vi "HFRR ADV v039.vi"() -> ()   [LabVIEW 2025] (continued)
  # "Calibration completed successfully. The measured stroke length is within the acceptable tolerance range of the factory calibration value."
  # "Calibration failed. The measured stroke length differs from the factory calibration value by more than 20%. Please perform the calibration again."
  # "Step 1 — Ball Holder"
  # "Remove the ball holder by loosening and removing the center screw for Friction calibration."
  # "Step 2 — Disc Holder"
  # "Remove the disc holder by loosening and removing the opposing screws. Clean any fluid present in the disc holder."
  # "Step 3 — Calibration Head"
  # "Place the calibration holder in position and securely tighten the center screw."
  # "Step 4 — Calibration Holder"
  # "Place the calibration holder in position and tighten the two securing screws"
  # "Step 5 — Tare (Spring at Free Length)"
  # "Ensure the spring is at its contact (compressed) length — the micrometer head is in contact. Click Tare Sensor to zero the friction force baseline."
  # "Step 6 — Measure Friction Force"
  # "Run the Actual Test to measure Friction Force."
  # "Spring Constant: k = 1.000 N/mm\nSpring force |F| = k Ч d"
  # "Calibrates the sample/bath temperature sensor. \nUsed for test specimen and lubricant temperature measurement."
  # "Calibrates the ambient air temperature sensor. \nUsed for environmental chamber monitoring."
  # "Set B\n60 °C\nHigh-point calibration"
  # "Set A\n0 °C\nIce-point calibration"
  # "Set B\n60 °C\nHigh-point calibration"
  # "Set A\n0 °C\nIce-point calibration"
  # "Select Temperature Sensor"
  # "Choose which temperature sensor you are calibrating. Both use the same two-\npoint procedure: 0 °C (ice-point) and 60 °C (high-point)."
  # "Step 1 — Reference Instrument Setup"
  # "Connect a calibrated reference to the DUT port. This calibration performs two sets: one at 0 °C and one at 60 °C."
  # "Set A\n0 °C\nIce-point calibration"
  # "Set B\n60 °C\nHigh-point calibration"
  # "Allow the temperature bath to stabilise for at least 2 minutes at each set-point before recording the reading."
  # "Step 2 — Set A:  0 °C Calibration"
  # "Connect the  0 °C reference connector. Wait for the temperature to stabilise. Once stable, and click Record Point."
  # "Step 3 — Set B:  60 °C Calibration"
  # "Connect the  60 °C reference connector. Wait for the temperature to stabilise. Once stable, and click Record Point."
  # "Sample Temperature Calibration Complete"
  # "Sample Temperature Calibration PASSED\nMax deviation 0.200 °C — within ±0.5 °C tolerance. Two-point correction applied (0 °C & 60 °C)."
  # "Sample  Temperature Calibration Failed\nmeasured Sample Temperature differs from the factory calibration value"
  # "Step 1 — Reference Instrument Setup"
  # "Connect a calibrated reference to the DUT port. This calibration performs two sets: one at 0 °C and one at 60 °C."
  # "Set A\n0 °C\nIce-point calibration"
  # "Set B\n60 °C\nHigh-point calibration"
  # "Allow the temperature bath to stabilise for at least 2 minutes at each set-point before recording the reading."
  # "Step 2 — Set A:  0 °C Calibration"
  # "Connect the  0 °C reference connector. Wait for the temperature to stabilise. Once stable, and click Record Point."
  # "Step 3 — Set B:  60 °C Calibration"
  # "Connect the  60 °C reference connector. Wait for the temperature to stabilise. Once stable, and click Record Point."
  # "Air Temperature Calibration Complete"
  # "Sample Temperature Calibration PASSED\nMax deviation 0.200 °C — within ±0.5 °C tolerance. Two-point correction applied (0 °C & 60 °C)."
  # "Sample  Temperature Calibration Failed\nmeasured Sample Temperature differs from the factory calibration value"
  # "System Control Commands\nS;1 - Starts the full automation cycle (Runs Priming-humidify till 70RH sequence first, then switches to Maintenance).\nS;0 - Stops the system immediately and enters Standby mode (Safe State: All actuators OFF).\nM;1 - Skips the priming sequence and jumps directly to Maintenance mode (PID control).\nR;1 - Resets the logic state machine and clears all errors, returning to Standby.\nService Mode (Manual Control)\nX;1 - Enters Manual Service Mode. This disables all automatic logic, sensor safety checks, and timers.\nX;0 - Exits Manual Service Mode and returns to Standby (Safe State).\nActuator Commands (Only work after sending X;1)\nP;[0-255] - Sets the Pump PWM. Note that this is Active Low (0 = Max Flow, 255 = Pump OFF).\nF;I;[0-255] - Sets the Intake Fan speed (0 = OFF, 255 = Max Speed).\nF;O;[0-255] - Sets the Exhaust Fan speed (0 = OFF, 255 = Max Speed).\nD;1 - Turns the Dehumidifier Relay ON.\nD;0 - Turns the Dehumidifier Relay OFF."
  # "%RH"
  # "ISO : WS1.4"
  # "Start test and end test log--- done\nDisable heater ON and Humidity ON during the test --- done\ntemprature and ---done\nhumidity reach log\nauto start run true logic and log\nmanual start log once"
  # "Reference Fluid Information"
  # "Note:\nMake sure to place all images in the folder \"C:\\WinDucom\\im\" before clicking on \"Import Image.\""
  # "NOTE:\nPlace all the images in the path \"C:\\WinDucom\\im\" before clicking on Import Image"
  # "Wear Scar Measurements"
  # "Reference Fluid Information"
  # "Graph :"
types:
  T1 = enum32{"Home", "Dashboard", "Imaging", "Report", "Analysis", "About", "Test Setup", "Advance", "Calibration"}
  T2 = enum32{"HOME", "Test Setup", "Acquire", "Adv Scar", "Adv Scar Report", "Compare Files", "Calibration", "About", "Advance", "Mooha"}
  T3 = enum16{"ASTM D6079", "ISO 12156", "CEC F-096-A-06", "Custom"}
  T4 = enum32{"Dashboard 1", "Dashboard 2", "Dashboard 3"}
  T5 = enum32{"COF", "Friction", "ECR", "Temperature", "Stroke"}
  T6 = enum32{"Coefficient Of Friction", "Air Temperature", "Humidity", "Stroke", "Sample Temperature", "Electrical Contact Resistance", "Frequency", "Air Temp vs Rh"}
  T7 = enum32{"Main", "Stroke", "Friction", "Temperature"}
  T8 = enum32{"Stroke Calibration", "Friction Force Calibration", "Temperature Calibration", "Default"}
  T9 = enum32{"Step 1", "Step 2", "Step 3", "Step 4", "Step 5", "Step 6", "Step 7", "Step 8", "Step 9"}
  T10 = enum32{"Test Progress", "Stroke Points Completed"}
  T11 = enum32{"Page 1", "Page 2", "Page 3", "Page 4", "Page 5", "Page 6", "Page 7"}
  T12 = enum32{"Main", "Step 1", "Step 2", "Step 3", "Step 4", "Air Step 1", "Air Step 2", "Air Step 3", "Air Step 4"}
  T13 = enum32{"Air Temperature", "Sample Temperature", "Default"}
  T14 = enum32{"COMMUNICATION", "CALIBRATION", "Temp Variables", "Camera", "WO 2465 (1)", "WO 2465 (2)", "WO 2465 (3)"}
  T15 = typedef "Auto Start enum.ctl" = enum16{"Init", "Humidity & Temperature On", "Reach point", "Maintain Stage", "Start Stage", "close", "Exit"}
  T16 = typedef "imagedata.ctl" = cluster{"image type":i32, "image depth":i32, "image":u8[], "mask":u8[], "colors":u32[], "Rectangle":cluster{"left":i16, "top":i16, "right":i16, "bottom":i16}}
  T17 = enum32{"HOME", "Test Setup", "Acquire", "Compare Files", "Print Report", "About", "Advance", "Mooha"}
  T18 = cluster{"Read Heave and Surge":string, "Bytes at Heave Port":dbl, "Heave and Surge COM Port:":refnum<visa-resource-name>, "Com Port 2":refnum<visa-resource-name>, "Residual Due":string, "Heave COM Status 2":bool, "Heave COM Status":bool, "Port 2":bool, "Sway PPR":dbl, "Surge PPR":dbl, "Heave PPR":dbl, "Sway Pitch":dbl, "Surge Pitch":dbl, "Heave Pitch":dbl, "Sway Pulses/mm":dbl, "Surge Pulses/mm":dbl, "Heave Pulses/mm":dbl, "inner loop":dbl, "Read Heave and Surge 2":string, "String 36":string, "Write S":bool, "WriteCC1":string[], "Heave COM Loop":i32, "LastCom":string, "EXIT":bool, "Error Heave":errorcluster}
  T19 = enum8{"Enabled", "Disabled", "Disabled and Grayed Out"}
  T20 = cluster{"Read Uno":string, "Bytes at Heave Port":dbl, "UNO COM Port:":refnum<visa-resource-name>, "UNO COM Port: 2":refnum<visa-resource-name>, "Residual Due":string, "UNO COM Status 2":bool, "UNO COM Status":bool, "Port 2":bool, "Sway PPR":dbl, "Surge PPR":dbl, "Heave PPR":dbl, "Sway Pitch":dbl, "Surge Pitch":dbl, "Heave Pitch":dbl, "Sway Pulses/mm":dbl, "Surge Pulses/mm":dbl, "Heave Pulses/mm":dbl, "inner loop":dbl, "Read Heave and Surge 2":string, "String 36":string, "Write S":bool, "WriteCC1":string[], "Heave COM Loop":i32, "LastCom":string, "EXIT":bool, "Error Heave":errorcluster}
  T21 = enum32{"HOME", "Test Setup", "Acquire", "Adv Scar", "Adv Scar Report", "Compare Files", "About", "Advance", "Mooha"}
  T22 = typedef "POST ANALYSIS ENUM.ctl" = enum16{"OPEN EXE", "INIT", "OPEN FILE", "FIT", "DRAW REC", "DRAW LINE", "PAN", "ZOOM IN", "ZOOM OUT", "SET ZOOM", "CLEAR ROI", "GET MEASUREMENTS", "RESIZE MODE", "STREAM START", "STREAM STOP", "SHOW UI", "MINIMIZE UI", "HIDE UI", "CKISE APP", "CLOSE CONNECTION", "SAVE IMAGE", "SET ROI COLOR", "READ", "TCP CHECK", "CLOSE"}
  T23 = typedef "CAMERA LIVE FEED ENUM.ctl" = enum16{"OPEN EXE", "INIT", "READ", "CAMERA CONNECT", "CAMERA START", "CAMERA STOP", "CAMERA GRAY", "CAMERA RGB", "CAMERA MINIMIZE", "CAMERA CLOSE", "CAMERA MODE LIST", "CAMERA MODE SET", "CAMERA RESTORE", "CAMERA SAVE", "CLOSE"}
  T24 = enum16{"Always On", "Always Off", "Off While Running"}
  T25 = enum32{"Page 1", "Page 2", "Page 3", "Page 4", "Page 5", "Page 6"}
  T26 = enum32{"Home", "Dashboard", "Imaging", "Report", "Analysis", "About", "Test Setup", "Advance"}
  T27 = cluster{"File Name":string, "Test Method":string, "Operator":string, "Fuel Description":string, "Date and time":string}
  T28 = enum32{"Home", "Dashboard", "Imaging", "Report", "Analysis", "About", "Test Setup"}
  T29 = enum32{"HOME", "Test Setup", "Acquire", "Compare Files", "About", "Advance", "Mooha"}
  T30 = typedef "NI_ReportGenerationCore.lvlib/HTML Report Image Alignment.ctl" = enum16{"(default)", "LEFT", "RIGHT", "TOP", "TEXTTOP", "MIDDLE", "ABSMIDDLE", "BASELINE", "BOTTOM", "ABSBOTTOM"}
  T31 = cluster{"y":dbl, "LVDT STROKE DISPLAY":dbl, "y":dbl}
  T32 = enum16{"INIT", "READ", "MANUAL WRITE", "WRITE", "CLOSE", "ERROR INIT"}
diagram:
  w3 = 0.0 ("ch0_filt")
  w5 = -9999999.0 ("max_ch0")
  w6 = 9999999.0 ("min_ch0")
  w17 = FALSE ("Visible")
  w18 = T19."Enabled" ("Disabled")
  w21 = FALSE ("Visible")
  w20 = FALSE ("Humidity Off Command")
  w36 = "" ("USER ID")
  (unwired) T21."HOME" ("Main Tab")
  # "Temperature Continue Air Step 2"
  # "[CH1]    - FF\n[CH2]   - TEMPERATURE\n[CH3]    - Humidity\n[CH4]    - AIR TEMP\n[CH5]\\- Visa Uno\n[CH6] \\- Visa Due\n[CH7]  \\- file path\n[CH8]   - Displacement Gain\n[CHA]   - Stroke Gain\n[CHB]   - Stroke PID Gain\n[CHC]   -Language Selection\n[CHD]   -Power +\n[CHE]   -Power_\n[CHF]   -Heater\n[CHG]   -Humidity Wet\n[CHH]   -Humidity Dry\n[CHI]   -Integral Time \n[CHIJ   -Air intercept\n[CHI]   -Temp Intercept"
  n1 = local write "Cal Password"("" ("Cal Password")) -> ()
  n2 = property on="Auto Start Test" class="Bool (strict)"("Visible"=TRUE) -> ()  [unwired: 2 in, 2 out]
  n3 = property on="FRICVALZ 2" class="Bool (strict)"("DisabledEnum"=w18) -> ()  [unwired: 2 in, 2 out]
  n4 = property on="FRICVALZ 4" class="Bool (strict)"("DisabledEnum"=w18) -> ()  [unwired: 2 in, 2 out]
  n5 = property on="FRICVALZ 3" class="Bool (strict)"("DisabledEnum"=w18) -> ()  [unwired: 2 in, 2 out]
  n6 = property on="About" class="Clust (strict)"("Visible"=FALSE) -> ()  [unwired: 2 in, 2 out]
  n7 = property on="Wrong Password" class="Str"("Visible"=w17) -> ()  [unwired: 2 in, 2 out]
  n8 = property on="Calibration 2" class="TabCtl (strict)"("Visible"=w17) -> ()  [unwired: 2 in, 2 out]
  n9 = flat-sequence {
    tunnel: [w63] -> w2
    tunnel: [w108] -> w28
    tunnel: w2 -> [w103]
    tunnel: [w109] -> w30
    tunnel: w28 -> [w109]
    tunnel: w30 -> [w169]
    tunnel: [w169] -> w29
    tunnel: w29 -> [w200]
    tunnel: [w200] -> w39
    tunnel: w39 -> [w207]
    tunnel: [w213] -> w27
    tunnel: [w201] -> w26
    tunnel: [w255] -> w1
    tunnel: [w254] -> _
    tunnel: w27 -> [w254]
    tunnel: w26 -> [w255]
    frame #0 {
      n10 = call "CLOSE CONNECTION.vi"("error in (no error)"="error in (no error) 2") -> ("error out"=w68:errorcluster)  [unwired: 10 in]
      n11 = call <vilib>:"Clear Errors.vi"("error in (no error)"=w68) -> ("error out"=w67:errorcluster)  [unwired: 5 in, 1 out]
      n12 = disable-structure shown="Enabled" {
        disable-tunnel: w67 -> [w95 _]
        disable-tunnel: [w94 _] -> w66
        frame Enabled {
          n13 = call <userlib>:"Fit VI window to Largest Dec.vi"("error in (no error)"=w95, "border spacing (2 px)"=1) -> ("error out"=w98:errorcluster, "dup VI Ref"=w102:refnum<vi>)  [unwired: 4 in]
          n14 = invoke on="Invoke Node" class="VI" method="FP.Run-Time Position.Maximized"(reference=w102, error in=w98) -> (error out=w99:errorcluster)  [unwired: 2 in, 3 out]
          n15 = call <vilib>:"Clear Errors.vi"("error in (no error)"=w99) -> ("error out"=w101:errorcluster)  [unwired: 5 in, 1 out]
          n16 = control-ref of="This VI"() -> (w93:refnum<vi>)
          n17 = invoke on="Invoke Node" class="VI" method="Default Vals.Reinit All"(reference=w93, error in=w101) -> (reference out=w97:refnum<vi>, error out=w96:errorcluster)  [unwired: 1 in, 1 out]
          n18 = Close Reference(reference=w97, error in (no error)=w96) -> (error out=w94:errorcluster)
        }
        frame Disabled {
        }
      }
      n19 = call "Stall Data Flow.vim"("value in"=w66, "milliseconds to wait"=u32 2000) -> ("value out"=w65:errorcluster)  [unwired: 1 out]
      n20 = call "Read Config.vi"("error in (no error)"=w65) -> ("error out"=w63:errorcluster, "STROKE PARAMETERS"=w74:dbl[], "ADC PARAMETERS"=w75:dbl[], "PID  PARAMETERS"=w76:dbl[], "CALIBRATION PARAMETERS"=w61:string[], "Stroke Calibration"=w73:string)  [unwired: 5 in]
      n21 = Index Array(array=w74) -> (element #1=w91:dbl, element #2=w92:dbl)  [unwired: 2 in]
      n22 = Index Array(array=w61) -> (element #1=w60:string, element #2=w59:string, element #3=w58:string, element #4=w57:string)  [unwired: 4 in]
      n23 = Index Array(array=w75) -> (element #1=w87:dbl, element #2=w88:dbl, element #3=w89:dbl, element #4=w90:dbl)  [unwired: 4 in]
      n24 = Index Array(array=w76) -> (element #1=w78:dbl, element #2=w79:dbl, element #3=w80:dbl, element #4=w81:dbl, element #5=w82:dbl, element #6=w83:dbl, element #7=w84:dbl, element #8=w85:dbl, element #9=w86:dbl)  [unwired: 9 in]
      n25 = local write "STROKE CALIBRATION"(w60) -> ()
      n26 = local write "FRICTION CALIBRATION"(w59) -> ()
      n27 = local write "TEMPERATURE CALIBRATION"(w58) -> ()
      n28 = Fract/Exp String To Number(string=w57) -> (number=w62:dbl)  [unwired: 3 in, 1 out]
      n29 = local write "milliseconds to wait"(w78) -> ()
      n30 = local write "dt"(w79) -> ()
      n31 = local write "kp"(w80) -> ()
      n32 = local write "ki"(w81) -> ()
      n33 = local write "kd"(w82) -> ()
      n34 = local write "max_step_change"(w83) -> ()
      n35 = local write "max_amplitude"(w84) -> ()
      n36 = local write "min_amplitude"(w85) -> ()
      n37 = local write "startup_cmd"(w86) -> ()
      n38 = local write "VREF"(w87) -> ()
      n39 = local write "ADC_Resolution"(w88) -> ()
      n40 = local write "PIEZO_CAL_FACTOR"(w89) -> ()
      n41 = local write "NORMAL_FORCE"(w90) -> ()
      n42 = local write "STROKE FILTER"(w91) -> ()
      n43 = local write "Add up Stroke"(w92) -> ()
      n44 = local write "Temperature diff"(w62) -> ()
      n45 = Spreadsheet String To Array(delimiter (Tab)=";", format string="", spreadsheet string=w73, array type (2D Dbl)=dbl[] []) -> (array=w77:dbl[])
      n46 = local write "calibration values"(w77) -> ()
    }
    frame #1 {
      n47 = property on="Auto Scar Check" class="Clust (strict)"("Visible"=TRUE) -> ()  [unwired: 2 in, 2 out]
      n48 = property on="Sign In" class="Bool (strict)"("DisabledEnum"=T19."Disabled" ("Disabled")) -> ()  [unwired: 2 in, 2 out]
      n49 = local write "sign in temp"(FALSE ("sign in temp")) -> ()
      n50 = call "dialog box.vi"("Status"="Before starting the test, verify that the microscope cable is connected.", "error in"=w103) -> ("error out"=w108:errorcluster)  [unwired: 8 in]
    }
    frame #2 {
      (unwired) TRUE ("Re-Initialise")
      # "kkkkk"
      # "C:\\Windows\\wndcm_pw_stdED hfrr.txt"
      # "C:\\LAB-IQ NXT"
      # "C:\\LAB-IQ NXT\\wndcm_pw_stdED hfrr.txt"
      # "password file"
      n51 = Current VI's Path() -> (path=w125:path)
      n52 = Strip Path(path=w125) -> (stripped path=w118:path)  [unwired: 1 out]
      n53 = local write "main tab sub"(enum32{"Page 1", "Page 2"}."Page 1" ("main tab sub")) -> ()
      n54 = local write "Main Tab Display"(T4."Dashboard 1" ("Main Tab Display")) -> ()
      n55 = local write "Main Tab"(T2."HOME" ("Main Tab")) -> ()
      n56 = Path To String(path=w118) -> (string=w120:string)
      n57 = Search/Split String(string=w120, search string/char (-)=".exe") -> (match + rest of string=w122:string)  [unwired: 1 in, 2 out]
      n58 = Match True/False String(2:".vi" ("false string"), 3:".exe" ("true string"), 4:w122) -> (0:w119:bool)  [unwired: 1 out]
      n59 = List Folder(path=path "C:/LAB-IQ" ("directory path"), pattern="*.txt") -> (filenames=w131:string[])  [unwired: 2 in, 3 out]
      n60 = case shown="True" w119 {
        tunnel: w118 -> [w140 w142]
        tunnel: [w140 w141] -> w116
        frame False {
        }
        frame True {
          n61 = Strip Path(path=w142) -> (stripped path=w141:path)  [unwired: 1 out]
        }
      }
      n62 = Search 1D Array(1D array=w131, element="wndcm_pw_stdED hfrr.txt") -> (index of element=w134:i32)  [unwired: 1 in]
      n63 = Equal?(x=w134, y=-1) -> (x = y?=w129:bool)
      n64 = Path To String(path=w116) -> (string=→"Gain path":string)
      n65 = case shown="True" w129 {
        frame False {
        }
        frame True {
          n66 = String To Byte Array(string="123\n") -> (unsigned byte array=w147:u8[])
          n67 = Array Size(array=w147) -> (size(s)=w146:i32)
          n68 = for {
            N: w146 -> [_]
            tunnel: w147 -> [w160]
            tunnel: [w157] -> w149 mode=indexing
            tunnel: w146 -> [w152]
            i -> [w150]
            n69 = Decrement(x=w152) -> (x-1=w153:i32)
            n70 = Index Array(array=w160, index=w150) -> (element=w159:u8)
            n71 = Equal?(x=w150, y=w153) -> (x = y?=w154:bool)
            n72 = Number To Decimal String(number=w159) -> (decimal integer string=w158:string)  [unwired: 1 in]
            n73 = Select(t="", s=w154, f="\r") -> (s? t:f=w151:string)
            n74 = Concatenate Strings(w158, w151) -> (w157:string)
          }
          n75 = local read "file path"() -> (w143:path)
          n76 = Concatenate Strings(w149) -> (w145:string)
          n77 = call <vilib>:"Write Characters To File.vi"("append to file? (new file:F)"=FALSE, "character string"=w145, "file path (dialog if empty)"=w143) -> ()  [unwired: 2 in, 1 out]
        }
      }
      n78 = local write "conststatus"(0.0 ("rpm value : 2")) -> ()
      n79 = local write "EVENT LOG"("") -> ()
      n80 = local write "COUNT"(0 ("COUNT")) -> ()
      n81 = local write "clk"(0.0 ("clk")) -> ()
      n82 = local write "Flag"(0.0 ("Flag")) -> ()
      n83 = local write "Lan flag"(0.0 ("Lan flag")) -> ()
      n84 = local write "Com flag"(u32 0 ("Com flag")) -> ()
      n85 = local write "refresh flag"(FALSE ("refresh flag")) -> ()
      "file path" <- path "C:/LAB-IQ/wndcm_pw_stdED hfrr.txt" ("file path")
      "FF buffer" <- dbl[] [] ("FF buffer")
    }
    frame #3 {
      # "C:\\WinDucom\\calibrate WO 2391.dcf"
      n86 = String To Path(string="C:\\LAB-IQ\\Image Calibrate v01.dcf") -> (path=w164:path)
      n87 = String To Path(string="C:\\LAB-IQ\\calibrate WO 2465.dcf") -> (path=w168:path)
      n88 = Open/Create/Replace File "Open File"(file path (use dialog)=w168) -> (refnum out=w167:refnum<file>)  [unwired: 5 in, 2 out]
      n89 = Open/Create/Replace File ("Open File")(file path (use dialog)=w164) -> (refnum out=w163:refnum<file>)  [unwired: 5 in, 2 out]
      n90 = for {
        N: 4 -> [_]
        tunnel: w163 -> [w175]
        i -> [w171]
        n91 = Read from Text File ("Read File")(file (use dialog)=w175) -> (text=w176:string)  [unwired: 3 in, 3 out]
        n92 = String Subset(string=w176, offset (0)=6, length (rest)=10 ("length (rest)")) -> (substring=w172:string)
        n93 = Fract/Exp String To Number(string=w172) -> (number=w170:dbl)  [unwired: 3 in, 1 out]
        n94 = case shown="3" w171 {
          tunnel: w170 -> [w177 w178 _ w179 _]
          frame 0 {
            n95 = local write "5x Gain"(w177) -> ()
          }
          frame 1 {
            n96 = local write "10x Gain"(w178) -> ()
          }
          frame 2 {
          }
          frame 3 {
            n97 = local write "100x gain"(w179) -> ()
          }
          frame 4, Default {
          }
        }
      }
      n98 = for {
        N: 24 -> [_]
        tunnel: w167 -> [w188]
        i -> [w182]
        (unwired) TRUE ("line mode (F)")
        n99 = Read from Text File "Read File"(file (use dialog)=w188) -> (text=w187:string)  [unwired: 3 in, 3 out]
        n100 = Match Pattern(string=w187, regular expression="]") -> (after substring=w185:string)  [unwired: 1 in, 3 out]
        n101 = String Subset(string=w187, offset (0)=5, length (rest)=10 ("length (rest)")) -> (substring=w180:string)
        n102 = Fract/Exp String To Number(string=w180) -> (number=w181:dbl)  [unwired: 3 in, 1 out]
        n103 = Match Pattern(string=w185, regular expression="-") -> (before substring=w183:string)  [unwired: 1 in, 3 out]
        n104 = case shown="18" w182 {
          tunnel: w181 -> [_ _ _ _ _ _ _ _ _ _ w195 _ _ _ _ _ _ _ _ _ _ _ _ _ _]
          tunnel: w183 -> [_ _ _ _ w191 w192 w193 _ _ _ _ _ _ _ _ _ _ _ _ _ w196 _ w197 w198 _]
          frame 0 {
          }
          frame 1 {
          }
          frame 2 {
          }
          frame 3 {
          }
          frame 4 {
            n105 = local write "Com Port 1"(w191) -> ()
          }
          frame 5 {
            n106 = local write "Com Port 2"(w192) -> ()
            n107 = local write "visa due"(w192) -> ()
          }
          frame 6 {
            n108 = String To Path(string=w193) -> (path=w194:path)
            n109 = local write "File Path"(w194) -> ()
          }
          frame 7 {
          }
          frame 8 {
          }
          frame 9 {
          }
          frame 10 {
            n110 = local write "Language Selection"(w195) -> ()
          }
          frame 11 {
          }
          frame 12 {
          }
          frame 13 {
          }
          frame 14 {
          }
          frame 15 {
          }
          frame 16 {
          }
          frame 17 {
          }
          frame 18 {
          }
          frame 21 {
          }
          frame 22 {
            n111 = local write "Com Port 3"(w196) -> ()
          }
          frame 23 {
          }
          frame 19 {
            n112 = local write "C3 :"(w197) -> ()
          }
          frame 20 {
            n113 = local write "Camera Port :"(w198) -> ()
          }
          frame 24, Default {
          }
        }
      }
    }
    frame #4 {
      n114 = Wait (ms)(milliseconds to wait=u32 1000) -> ()  [unwired: 1 out]
    }
    frame #5 {
      w216 = u32 2000 ("milliseconds to wait")
      w243 = u32 2000 ("milliseconds to wait")
      n115 = call "CAMERA LIVE FEED FGV.vi"("Enum - Menu"=CAMERA_LIVE_FEED_ENUM."OPEN EXE", "error in (no error)"=w207) -> ("error out"=w249:errorcluster)  [unwired: 8 in, 1 out]
      n116 = call "IMAGE ANALYSIS.vi"("Enum"=POST_ANALYSIS_ENUM."OPEN EXE", "error in"=w207) -> ("error out"=w204:errorcluster)  [unwired: 8 in, 1 out]
      n117 = call "Stall Data Flow.vim"("value in"=w249, "milliseconds to wait"=w243) -> ("value out"=w247:errorcluster)  [unwired: 1 out]
      n118 = call "Stall Data Flow.vim"("value in"=w204, "milliseconds to wait"=u32 8000) -> ("value out"=w203:errorcluster)  [unwired: 1 out]
      n119 = call "CAMERA LIVE FEED FGV.vi"("Enum - Menu"=CAMERA_LIVE_FEED_ENUM."INIT", "error in (no error)"=w247) -> ("error out"=w245:errorcluster)  [unwired: 8 in, 1 out]
      n120 = call "IMAGE ANALYSIS.vi"("Enum"=POST_ANALYSIS_ENUM."INIT", "error in"=w203) -> ("error out"=w201:errorcluster)  [unwired: 8 in, 1 out]
      n121 = case shown="Error .." w245 {
        selector: w245 -> [w250 _]
        tunnel: [w250 _] -> w244
        frame No Error {
        }
        frame Error {
          n122 = One Button Dialog(message="Camera initialization error.\nPlease Restart the software") -> ()  [unwired: 1 in, 1 out]
        }
      }
      n123 = property on="Camera Port :" class="CmbBox"() -> ("Strings[]"=w241:string[], "Value"=w242:string)  [unwired: 2 in, 2 out]
      n124 = Search 1D Array(1D array=w241, element=w242) -> (index of element=w240:i32)  [unwired: 1 in]
      n125 = Type Cast(type=30, x=w240) -> (*(type *) &x=w238:i32)
      n126 = call "Stall Data Flow.vim"("value in"=w244, "milliseconds to wait"=w243) -> ("value out"=w220:errorcluster)  [unwired: 1 out]
      n127 = Add(x=w238, y=48) -> (x+y=w219:i32)
      n128 = call "CAMERA LIVE FEED FGV.vi"("Enum - Menu"=CAMERA_LIVE_FEED_ENUM."CAMERA CONNECT", "error in (no error)"=w220, "CAMERA PORT"=w219) -> ("error out"=w229:errorcluster)  [unwired: 7 in, 1 out]
      n129 = call "Stall Data Flow.vim"("value in"=w229, "milliseconds to wait"=u32 5000) -> ("value out"=w230:errorcluster)  [unwired: 1 out]
      n130 = call "CAMERA LIVE FEED FGV.vi"("Enum - Menu"=CAMERA_LIVE_FEED_ENUM."CAMERA MODE LIST", "error in (no error)"=w230) -> ("error out"=w232:errorcluster)  [unwired: 8 in, 1 out]
      n131 = call "Stall Data Flow.vim"("value in"=w232, "milliseconds to wait"=w216) -> ("value out"=w231:errorcluster)  [unwired: 1 out]
      n132 = call "CAMERA LIVE FEED FGV.vi"("Enum - Menu"=CAMERA_LIVE_FEED_ENUM."READ", "error in (no error)"=w231) -> ("error out"=w218:errorcluster, "data out"=→"Camera List":string)  [unwired: 8 in]
      n133 = Type Cast(type=30, x=0) -> (*(type *) &x=w212:i32)
      n134 = call "Stall Data Flow.vim"("value in"=w218, "milliseconds to wait"=w216) -> ("value out"=w217:errorcluster)  [unwired: 1 out]
      n135 = Add(x=w212, y=48) -> (x+y=w210:i32)
      n136 = call "CAMERA LIVE FEED FGV.vi"("Enum - Menu"=CAMERA_LIVE_FEED_ENUM."CAMERA MODE SET", "error in (no error)"=w217, "CAMERA MODE"=w210) -> ("error out"=w214:errorcluster)  [unwired: 7 in, 1 out]
      n137 = call "Stall Data Flow.vim"("value in"=w214, "milliseconds to wait"=u32 2000) -> ("value out"=w234:errorcluster)  [unwired: 1 out]
      n138 = call "CAMERA LIVE FEED FGV.vi"("Enum - Menu"=CAMERA_LIVE_FEED_ENUM."CAMERA START", "error in (no error)"=w234) -> ("error out"=w235:errorcluster)  [unwired: 8 in, 1 out]
      n139 = call "Stall Data Flow.vim"("value in"=w235, "milliseconds to wait"=u32 1000) -> ("value out"=w236:errorcluster)  [unwired: 1 out]
      n140 = call "CAMERA LIVE FEED FGV.vi"("Enum - Menu"=CAMERA_LIVE_FEED_ENUM."CAMERA MINIMIZE", "error in (no error)"=w236) -> ("error out"=w213:errorcluster)  [unwired: 8 in, 1 out]
    }
    frame #6 {
      n141 = case shown="No Error" w254 {
        frame No Error {
          n142 = property on="Auto Scar Check" class="Clust (strict)"("Visible"=FALSE) -> ()  [unwired: 2 in, 2 out]
        }
        frame Error {
        }
      }
      n143 = property on="Sign In" class="Bool (strict)"("DisabledEnum"=T19."Enabled" ("Disabled")) -> ()  [unwired: 2 in, 2 out]
      n144 = local write "sign in temp"(TRUE ("sign in temp")) -> ()
    }
  }
  n145 = local write "SCAR MEASURMENT"(enum32{"Auto Scar", "Manual Scar"}."Manual Scar" ("SCAR MEASURMENT")) -> ()
  n146 = local write "Temperature Off Command"(w20) -> ()
  n147 = local write "Main Dashboard Buttons"(T1."Home" ("Main Dashboard Buttons")) -> ()
  n148 = local write "Humidity Off Command"(w20) -> ()
  n149 = local write "CAMERA ROI MIN TEMP"(w20) -> ()
  n150 = local write "TEST FILE NAM,E SAVED"(w20) -> ()
  n151 = local write "LIVE FEED MIN TEMP"(w20) -> ()
  n152 = local write "SCAR MEASURMENT"(enum32{"Auto Scar", "Manual Scar"}."Manual Scar" ("SCAR MEASURMENT")) -> ()
  n153 = local write "Auto stop temp"(w21) -> ()
  n154 = local write "main tab sub"(enum32{"Page 1", "Page 2"}."Page 1" ("main tab sub")) -> ()
  n155 = while {
    stop <- w266 stop-if-true
    (unwired) string[] ["STROKE CALIBRATION", "FRICTION CALIBRATION", "TEMPERATURE CALIBRATION", "TEMPERATURE DIFF VALUE"]
    n156 = local read "Ambient Temperature"() -> (w264:dbl)
    n157 = local read "Sample Temperature"() -> (w263:dbl)
    n158 = Wait (ms)(milliseconds to wait=u32 200) -> ()  [unwired: 1 out]
    n159 = local write "Sensor value"(w264) -> ()
    n160 = local write "Sensor value"(w264) -> ()
    n161 = local write "Sensor value"(w263) -> ()
    n162 = local write "Sensor value"(w263) -> ()
    n163 = local write "Temperature — Live (Set A: 0 °C)"(w264) -> ()
    n164 = local write "Temperature — Live (Set A: 60 °C)"(w264) -> ()
    n165 = local write "Temperature — Live (Set A: 60 °C)"(w263) -> ()
    n166 = local write "Temperature — Live (Set A: 0 °C)"(w263) -> ()
    n167 = case shown="True" "Save Button" {
      selector: "Save Button" -> [_ w306]
      frame False {
      }
      frame True {
        n168 = local read "Temperature diff"() -> (w302:dbl)
        n169 = Not(x=w306) -> (.not. x?=w305:bool)
        n170 = local read "milliseconds to wait"() -> (w338:u32)
        n171 = local read "max_step_change"() -> (w343:dbl)
        n172 = local read "max_amplitude"() -> (w344:dbl)
        n173 = local read "min_amplitude"() -> (w345:dbl)
        n174 = local read "PIEZO_CAL_FACTOR"() -> (w349:dbl)
        n175 = local write "Save Button"(w305) -> ()
        n176 = local read "startup_cmd"() -> (w346:dbl)
        n177 = local read "NORMAL_FORCE"() -> (w350:dbl)
        n178 = local read "ADC_Resolution"() -> (w348:dbl)
        n179 = local read "calibration values"() -> (w353:dbl[])
        n180 = local read "kp"() -> (w340:dbl)
        n181 = local read "kd"() -> (w342:dbl)
        n182 = local read "dt"() -> (w339:dbl)
        n183 = local read "ki"() -> (w341:dbl)
        n184 = local read "STROKE FILTER"() -> (w351:i32)
        n185 = local read "Add up Stroke"() -> (w352:dbl)
        n186 = Number To Fractional String(number=w302) -> (F-format string=w301:string)  [unwired: 3 in]
        n187 = local read "VREF"() -> (w347:dbl)
        n188 = Insert Into Array(array=string[] [], new element #1="STROKE CALIBRATION", new element #2="FRICTION CALIBRATION", new element #3="TEMPERATURE CALIBRATION", new element #4=w301) -> (w303:string[])  [unwired: 1 in]
        n189 = Insert Into Array(array=dbl[] [], new element #1=w338, new element #2=w339, new element #3=w340, new element #4=w341, new element #5=w342, new element #6=w343, new element #7=w344, new element #8=w345, new element #9=w346) -> (w354:dbl[])  [unwired: 1 in]
        n190 = Insert Into Array(array=dbl[] [], new element #1=w347, new element #2=w348, new element #3=w349, new element #4=w350) -> (w355:dbl[])  [unwired: 1 in]
        n191 = Array To Spreadsheet String(delimiter (Tab)=";", array=w353, 3:"" ("format string")) -> (spreadsheet string=w357:string)
        n192 = Insert Into Array(array=dbl[] [], new element #1=w351, new element #2=w352) -> (w356:dbl[])  [unwired: 1 in]
        n193 = call "Write Config.vi"("Stroke Calibration"=w357, "CALIBRATION PARAMETERS"=w303, "STROKE PARAMETERS"=w356, "ADC PARAMETERS"=w355, "PID  PARAMETERS"=w354) -> ("error out"=w336:errorcluster)  [unwired: 6 in]
        n194 = call "Stall Data Flow.vim"("value in"=w336, "milliseconds to wait"=u32 2000) -> ("value out"=w337:errorcluster)  [unwired: 1 out]
        n195 = call "Read Config.vi"("error in (no error)"=w337) -> ("STROKE PARAMETERS"=w334:dbl[], "ADC PARAMETERS"=w333:dbl[], "PID  PARAMETERS"=w332:dbl[], "CALIBRATION PARAMETERS"=w297:string[], "Stroke Calibration"=w335:string)  [unwired: 5 in, 1 out]
        n196 = Index Array(array=w332) -> (element #1=w330:dbl, element #2=w329:dbl, element #3=w328:dbl, element #4=w327:dbl, element #5=w326:dbl, element #6=w325:dbl, element #7=w324:dbl, element #8=w323:dbl, element #9=w322:dbl)  [unwired: 9 in]
        n197 = Index Array(array=w333) -> (element #1=w321:dbl, element #2=w320:dbl, element #3=w319:dbl, element #4=w318:dbl)  [unwired: 4 in]
        n198 = Index Array(array=w334) -> (element #1=w317:dbl, element #2=w316:dbl)  [unwired: 2 in]
        n199 = Index Array(array=w297) -> (element #1=w294:string, element #2=w293:string, element #3=w292:string, element #4=w296:string)  [unwired: 4 in]
        n200 = Spreadsheet String To Array(delimiter (Tab)=";", format string="", spreadsheet string=w335, array type (2D Dbl)=dbl[] []) -> (array=w331:dbl[])
        n201 = local write "VREF"(w321) -> ()
        n202 = local write "ADC_Resolution"(w320) -> ()
        n203 = local write "PIEZO_CAL_FACTOR"(w319) -> ()
        n204 = local write "NORMAL_FORCE"(w318) -> ()
        n205 = local write "STROKE CALIBRATION"(w294) -> ()
        n206 = local write "FRICTION CALIBRATION"(w293) -> ()
        n207 = local write "TEMPERATURE CALIBRATION"(w292) -> ()
        n208 = Fract/Exp String To Number(string=w296) -> (number=w295:dbl)  [unwired: 3 in, 1 out]
        n209 = local write "STROKE FILTER"(w317) -> ()
        n210 = local write "Add up Stroke"(w316) -> ()
        n211 = local write "calibration values"(w331) -> ()
        n212 = local write "milliseconds to wait"(w330) -> ()
        n213 = local write "dt"(w329) -> ()
        n214 = local write "kp"(w328) -> ()
        n215 = local write "ki"(w327) -> ()
        n216 = local write "kd"(w326) -> ()
        n217 = local write "max_step_change"(w325) -> ()
        n218 = local write "max_amplitude"(w324) -> ()
        n219 = local write "min_amplitude"(w323) -> ()
        n220 = local write "startup_cmd"(w322) -> ()
        n221 = local write "Temperature diff"(w295) -> ()
      }
    }
    n222 = local read "USER ID"() -> (w261:string)
    n223 = local read "run test Calibration"() -> (w259:bool)
    n224 = disable-structure shown="Enabled" {
      disable-tunnel: [w267 w278] -> w260
      frame Disabled {
        n225 = local read "Point 1 - 0.2 mm"() -> (w277:bool)
        n226 = local read "Point 2 - 0.4 mm"() -> (w276:bool)
        n227 = local read "Point 3 - 0.6 mm"() -> (w275:bool)
        n228 = local read "Point 4 - 0.8 mm"() -> (w274:bool)
        n229 = local read "Point 5 - 1.0 mm"() -> (w273:bool)
        n230 = local read "Point 6 - 1.2 mm"() -> (w272:bool)
        n231 = And(x=w277, y=w276) -> (x .and. y?=w271:bool)
        n232 = And(x=w275, y=w274) -> (x .and. y?=w270:bool)
        n233 = And(x=w273, y=w272) -> (x .and. y?=w268:bool)
        n234 = And(x=w271, y=w270) -> (x .and. y?=w269:bool)
        n235 = And(x=w269, y=w268) -> (x .and. y?=w267:bool)
      }
      frame Enabled {
        n236 = local read "Point 5 - 1.0 mm"() -> (w278:bool)
      }
    }
    n237 = local read "START TEMP"() -> (w258:bool)
    n238 = local write "tested by 2"(w261) -> ()
    n239 = And(x=w258, y=w259) -> (x .and. y?=w257:bool)
    n240 = case shown="True" w257 {
      frame False {
        w279 = TRUE ("PAUSE")
        n241 = call "ELAPSED TIMER VI - Calibration.vi"("RESET"=w279, "PAUSE"=w279) -> ()  [unwired: 7 in, 3 out]
      }
      frame True {
        w282 = FALSE ("PAUSE")
        n242 = call "ELAPSED TIMER VI - Calibration.vi"("TARGET"=60.0, "RESET"=w282, "PAUSE"=w282) -> ("ELAPSED INDICATION"=w280:bool)  [unwired: 6 in, 2 out]
        n243 = case shown="True" w280 {
          frame False {
          }
          frame True {
            n244 = stacked-sequence {
              frame #0 {
                n245 = local write "START TEMP"(FALSE ("START TEMP")) -> ()
              }
              frame #1 {
                n246 = Wait (ms)(milliseconds to wait=u32 1500) -> ()  [unwired: 1 out]
              }
              frame #2 {
                n247 = local write "Due Write"("VC;0") -> ()
              }
              frame #3 {
                n248 = Wait (ms)(milliseconds to wait=u32 1500) -> ()  [unwired: 1 out]
              }
              frame #4 {
                n249 = local write "Due Write"("VC;0") -> ()
              }
            }
          }
        }
      }
    }
    n250 = case shown="False" w260 {
      frame False {
        n251 = property on="Accept & Save" class="Bool (strict)"("DisabledEnum"=T19."Disabled" ("Disabled")) -> ()  [unwired: 2 in, 2 out]
        n252 = property on="Tab Control 5" class="TabCtl (strict)"("Value"=enum32{"OK", "NG"}."NG" ("Tab Control 5")) -> ()  [unwired: 2 in, 2 out]
      }
      frame True {
        n253 = property on="Accept & Save" class="Bool (strict)"("DisabledEnum"=T19."Enabled" ("Disabled")) -> ()  [unwired: 2 in, 2 out]
        n254 = property on="Tab Control 5" class="TabCtl (strict)"("Value"=enum32{"OK", "NG"}."OK" ("Tab Control 5")) -> ()  [unwired: 2 in, 2 out]
      }
    }
    n255 = local read "Quit"() -> (w266:bool)
  }
  n256 = local write "USERNAME"(w36) -> ()
  n257 = local write "Main Tab"(T2."HOME" ("Main Tab")) -> ()
  n258 = local write "USER ID"(w36) -> ()
  n259 = property on="Auto Scar Check  2" class="Clust (strict)"("Visible"=w21) -> (error out=w24:errorcluster)  [unwired: 2 in, 1 out]
  n260 = property on="Quit" class="Bool (strict)"("Value"=FALSE ("Quit")) -> (error out=w38:errorcluster)  [unwired: 2 in, 1 out]
  n261 = while {
    stop <- w358 stop-if-true
    n262 = event shown="[41] \"Temperature Continue Step 6\": Value Change" {
      selector: _ -> [_ _ _ _ _ _ _ _ _ _ _ _ _ _ _ _ _ _ _ _ _ _ _ _ _ _ _ _ _ _ _ _ _ _ _ _ _ _ _ _ _ _ _ _ _ _ _ _ _ _ _]
      dyn-events: _ -> [_ _ _ _ _ _ _ _ _ _ _ _ _ _ _ _ _ _ _ _ _ _ _ _ _ _ _ _ _ _ _ _ _ _ _ _ _ _ _ _ _ _ _ _ _ _ _ _ _ _ _]
      timeout: 100 -> [_ _ _ _ _ _ _ _ _ _ _ _ _ _ _ _ _ _ _ _ _ _ _ _ _ _ _ _ _ _ _ _ _ _ _ _ _ _ _ _ _ _ _ _ _ _ _ _ _ _ _]
      tunnel: [FALSE FALSE FALSE _ FALSE _ _ _ _ _ _ _ _ _ _ _ _ _ _ _ _ _ _ _ _ _ _ _ _ _ _ _ _ _ _ _ _ _ _ _ _ _ _ _ _ _ _ _ _ _ TRUE] -> w358
      event Timeout {
        n263 = event-data() -> ()  [unwired: 1 in, 3 out]
        n264 = disable-structure shown="Disabled" {
          frame Disabled {
            n265 = local read "Auto Start Test"() -> (w372:bool)
            n266 = local read "RUN"() -> (w373:bool)
            n267 = Or(x=w373, y=w372) -> (x .or. y?=w371:bool)
            n268 = case shown="True" w371 {
              frame False {
                w374 = TRUE ("PAUSE")
                n269 = call "ELAPSED TIMER VI - abort test.vi"("RESET"=w374, "PAUSE"=w374) -> ()  [unwired: 7 in, 3 out]
              }
              frame True {
                n270 = local read "Stroke 2"() -> (w379:dbl)
                n271 = local read "FF 3"() -> (w381:dbl)
                n272 = Equal?(x=w379, y=0.95 ("Stroke 2")) -> (x = y?=w376:bool)
                n273 = Equal?(x=w381, y=0.0 ("FF 3")) -> (x = y?=w377:bool)
                n274 = Or(x=w377, y=w376) -> (x .or. y?=w375:bool)
                n275 = case shown="True" w375 {
                  selector: w375 -> [_ w386]
                  frame False {
                    w382 = TRUE ("PAUSE")
                    n276 = call "ELAPSED TIMER VI - abort test.vi"("RESET"=w382, "PAUSE"=w382) -> ()  [unwired: 7 in, 3 out]
                  }
                  frame True {
                    n277 = Not(x=w386) -> (.not. x?=w385:bool)
                    n278 = call "ELAPSED TIMER VI - abort test.vi"("TARGET"=60.0, "RESET"=w385, "PAUSE"=FALSE) -> ("ELAPSED INDICATION"=w383:bool)  [unwired: 6 in, 2 out]
                    n279 = case shown="True" w383 {
                      frame False {
                      }
                      frame True {
                        n280 = stacked-sequence {
                          frame #0 {
                            w388 = FALSE
                            n281 = local write "RUN"(w388) -> ()
                            n282 = local write "Auto Start Test"(w388) -> ()
                          }
                          frame #1 {
                            n283 = One Button Dialog(message="Test stopped due to a communication error. Reconnect the C1 and C2 cables.") -> ()  [unwired: 1 in, 1 out]
                          }
                        }